vi "UHR-Fleezers Control (host) - Avogadro v2.vi"() -> ()   [LabVIEW 2014] (continued)
0.06928382213812578, 0.06928028199102658, 0.06922544022949823, 0.06920560319833882, 0.06922019104586834, 0.06924063844721727, 0.06926700643940453, 0.06926718955046138, 0.06929898983733536, 0.06925055696279696, 0.06931403546250704, 0.0692955107272551, 0.06922473830378026, 0.06928565324869435, 0.06928879665517038, 0.06925675222022058, 0.06923380230109463, 0.06924164555802997, 0.06928174687948142, 0.06932566301461739, 0.06929343546861073, 0.06929117709890951, 0.06922135074922843, 0.06925714896084378, 0.06925159459211913, 0.06932630390331637, 0.0692147892696911, 0.0692787255470433, 0.06924900051881369, 0.06927286599322391, 0.06931833857234315, 0.06929380169072444, 0.06926581621753496, 0.06930823694570659, 0.06927799310281588, 0.06928147221289614, 0.06926407666249483, 0.06927030243842792, 0.06922562334055508, 0.06926313058870108, 0.06927741325113584, 0.06928653828546916, 0.0692268440809341, 0.06926950895718155, 0.06926767784661299, 0.06920160527359746, 0.06925424970244355, 0.06928284554582255, 0.06921207312234773, 0.06924927518539896, 0.06922894985808796, 0.0692571184423343, 0.06920566423535776, 0.06925980407116819, 0.06928257087923728, 0.06927216406750597, 0.06922339548936332, 0.06926215399639785, 0.06920325327310915, 0.06924637592699874, 0.06921677297280703, 0.06922513504440345, 0.06916922513504342, 0.06923242896816821, 0.06922205267494637, 0.06921817682424293, 0.06918747520371007, 0.06919815668202667, 0.06919797357096982, 0.06923786126285494, 0.06921915341654616, 0.06922568437757402, 0.06918127994628644, 0.06922547074800768, 0.06924582659382818, 0.06921549119540904, 0.0692108218634592, 0.06915109714041469, 0.06908627582628768, 0.06918482009338565, 0.0691833857234403, 0.06921112704855398, 0.06916605121005792, 0.06920618305001885, 0.069132267220068, 0.06920310068056178, 0.06923773918881705, 0.06922501297036555, 0.0691231116672252, 0.06918146305734331, 0.06919553209021173, 0.06922956022827748, 0.06919336527603893, 0.06926355784783372, 0.06923966185491404, 0.06929560228278353, 0.06927195043793963, 0.06928467665639111, 0.06924256111331427, 0.06929725028229522, 0.06923395489364202, 0.06924204229865316, 0.06922525711844135, 0.06924771874141569, 0.06915643787957299, 0.06924536881618604, 0.06916010010071011, 0.06918335520493081, 0.06919299905392522, 0.06916858424634442, 0.06912195196386511, 0.06918533890804675, 0.06917004913479928, 0.0691453596606332, 0.06913382366405128, 0.06916522721030208, 0.06916882839442023, 0.06921610156559856, 0.06917017120883717, 0.0692243110446476, 0.06924466689046808, 0.06922168645283266, 0.06920572527237671, 0.06918127994628644, 0.06914984588152617, 0.06918936735129759, 0.06918237861262758, 0.0692385631885729, 0.06924268318735215, 0.06924527726065761, 0.06918936735129759, 0.06917838068788623, 0.0691982482375551, 0.06920844141972009, 0.06918158513138122, 0.06920218512527751, 0.06922443311868551, 0.06925321207312136, 0.06926328318124844, 0.06932975249488717, 0.0693037812433231, 0.06932642597735428, 0.06933487960447914, 0.0693373516037467, 0.06928443250831531, 0.0693576769310577, 0.06930802331614026, 0.06936115604113798, 0.06934812463759171, 0.06937299722281466, 0.06932422864467201, 0.0693681142612985, 0.06933906064027735, 0.0693524582659373, 0.06936597796563516, 0.06941334269234192, 0.0694059877315582, 0.0694610431226529, 0.06942216254158048, 0.06946394238105313, 0.06943000579851583, 0.06939817499313235, 0.06938685262611675, 0.06938254951628064, 0.06940998565629956, 0.06944059572130398, 0.06940183721426947, 0.06945286416211334, 0.06943455305642773, 0.06941611987670424, 0.06938065736869313, 0.06938911099581799, 0.06940125736258942, 0.06936140018921379, 0.06936152226325168, 0.06936069826349583, 0.06934803308206329, 0.06941767632068752, 0.06940769676808886, 0.06943382061220031, 0.06938242744224274, 0.06941331217383244, 0.06935120700704879, 0.06939872432630292, 0.06936268196661176, 0.06943717764824267, 0.06937897885067196, 0.06938016907254152, 0.06935740226447241, 0.0693983581041892, 0.06941715750602642, 0.0694203619495214, 0.06937653736991388, 0.06944013794366186, 0.0693949400311279, 0.06943995483260498, 0.06938178655354375, 0.0694314096499517, 0.06938126773888265, 0.06940684224982353, 0.06935407574693954, 0.06939741203039546, 0.06940458388012231, 0.06944648579363286, 0.06942982268745895, 0.06944026001769976, 0.06939869380779344, 0.0694128543961903, 0.06941743217261172, 0.0694466689046897, 0.06944306772057154, 0.06944724875636975, 0.0693813287759016, 0.0694225287636942, 0.06942335276345005, 0.06942286446729842, 0.06936649678029627, 0.06939878536332188, 0.06938465529343447, 0.06938209173863849, 0.06943617053742997, 0.06940986358226166, 0.0693832514419986, 0.06940720847193725, 0.06944444105349797, 0.06941395306253144, 0.06938648640400304, 0.0693665883358247, 0.06930732139042231, 0.0692876369518103, 0.06930552079836323, 0.06935331278420263, 0.0692883999145472, 0.06935364848780687, 0.06931913205358953, 0.06933057649464301, 0.06932050538651595, 0.0692761925107568, 0.0693024994659251, 0.06931672109134092, 0.06930591753898642, 0.06935569322794176, 0.06926532792138335, 0.06928382213812578, 0.06927756584368322, 0.06927701651051264, 0.06923596911526743, 0.06926230658894522, 0.06935776848658613, 0.06929181798760851, 0.06931965086825062, 0.06932584612567425, 0.06934714804528849, 0.06931525620288607, 0.06937565233313907, 0.06932847071748918, 0.06936109500411901, 0.06931763664662519, 0.0692788476210812, 0.06924845118564311, 0.06926844080934988, 0.06921359904782153, 0.06921311075166992, 0.06931092257454047, 0.0693307290871904, 0.06935657826471657, 0.06931730094302097, 0.0693545030060722, 0.06926172673726516, 0.06934031189916587, 0.06935810419019038, 0.06938956877346013, 0.06931397442548808, 0.06935932493056941, 0.06935944700460732, 0.06934925382244232, 0.06938404492324496, 0.06937766655476449, 0.06930881679738664, 0.06933249916074001, 0.06928376110110684, 0.06932816553239442, 0.06931122775963525, 0.06934678182317477, 0.06935254982146573, 0.06938245796075221, 0.06937485885189269, 0.06939579454939322, 0.06931440168462075, 0.06936371959593396, 0.06932306894131193, 0.06934836878566752, 0.0693476363414401, 0.06934827723013909, 0.06930079042939444, 0.06931440168462075, 0.06926267281105893, 0.06928592791527964, 0.0692700888088616, 0.06928601947080806, 0.06929694509720048, 0.06930405590990837, 0.06929740287484261, 0.06930442213202209, 0.06922742393261415, 0.06928464613788164, 0.0692596514786208, 0.06930793176061184, 0.069199652088991, 0.06925479903561411, 0.06921405682546367, 0.06921103549302554, 0.0692374340037223, 0.0692571184423343, 0.06916357921079036, 0.06923007904293857, 0.06926007873775347, 0.06929618213446358, 0.06919635608996759, 0.06923010956144804, 0.06919727164525186, 0.06923825800347815, 0.06919989623706681, 0.06925031281472116, 0.06920294808801442, 0.06928122806482033, 0.06922745445112363, 0.06929078035828631, 0.06922525711844137, 0.06926862392040675, 0.06922998748741013, 0.06929773857844684, 0.06921878719443245, 0.0692302926725049, 0.06921588793603223, 0.06924692526016932, 0.06919693594164764, 0.0692117374187435, 0.06916132084108916, 0.0692548295541236, 0.06917160557878256, 0.06922321237830648, 0.06927637562181364, 0.06926190984832203, 0.06919534897915489, 0.0692418591875963, 0.06920361949522287, 0.06919110690633773, 0.06915567491683608, 0.06916843165379705, 0.06909604174932, 0.0691276894436466, 0.06915414899136228, 0.06914127018036341, 0.06910113834040249, 0.06911123996703905, 0.0691143528550056, 0.06914590899380377, 0.06910333567308476, 0.06913177892391639, 0.0690913418988607, 0.06912509537034113, 0.06914682454908805, 0.06910397656178374, 0.06911520737327093, 0.06913068025757525, 0.06910980559709366, 0.06910458693197327, 0.06907867671742815, 0.06909610278633894, 0.06905011139255862, 0.06911847285378485, 0.0691039155247648, 0.0691266823328339, 0.06910153508102568, 0.06914807580797655, 0.06916101565599438, 0.06917352824487955, 0.06917227698599103, 0.0691720633564247, 0.06911679433576366, 0.06917352824487955, 0.06914658040101224, 0.06918637653736893, 0.06920084231086056, 0.06919824823755509, 0.06915613269447822, 0.06918848231452278, 0.06918335520493081, 0.06919895016327304, 0.06913116855372686, 0.0691971190527045, 0.06918787194433326, 0.06919757683034664, 0.06918262276070339, 0.06924823755607679, 0.06920020142216156, 0.06926316110721055, 0.06924225592821949, 0.06923294778282932, 0.06919544053468331, 0.06923789178136441, 0.06921427045503001, 0.06923743400372227, 0.06922196111941795, 0.06923917355876243, 0.06915729239783831, 0.06921027253028865, 0.06919714957121396, 0.0692110965300445, 0.06918735312967217, 0.06918729209265322, 0.06915085299233888, 0.06920081179235107, 0.06917542039246705, 0.06917288735618055, 0.0691332743308807, 0.06919083223975243, 0.06917096469008356, 0.06918506424146147, 0.06919516586809803, 0.06922379222998651, 0.06913037507248047, 0.06924118778038783, 0.06920123905148376, 0.06923831904049708, 0.06914429151280153, 0.06924344615008905, 0.06921396526993524, 0.06924512466811023, 0.06916586809900106, 0.06923044526505227, 0.0691588488418216, 0.06921011993774126, 0.06913885921811481, 0.06914893032624188, 0.0691214636677135, 0.06917664113284609, 0.06917542039246706, 0.06919003875850606, 0.0692187261574135, 0.06922055726798206, 0.06918701742606793, 0.06921475875118162, 0.06920477919858296, 0.06921805475020502, 0.06920517593920615, 0.06922910245063534, 0.06923438215277468, 0.06924124881740677, 0.06926117740409461, 0.06928516495254274, 0.06921857356486612, 0.06925373088778247, 0.06925061799981592, 0.06924826807458626, 0.0692750328073967, 0.06931464583269656, 0.06937162388988824, 0.06935654774620709, 0.06929197058015589, 0.06936548966948355, 0.0693017365031882, 0.06939542832727952, 0.06935874507888937, 0.06938279366435644, 0.06938038270210783, 0.06944230475783464, 0.06940006714071986, 0.06944495986815905, 0.06940940580461952, 0.0694348582415225, 0.06944514297921592, 0.0694868617816696, 0.06947965941343326, 0.06947242652668745, 0.06950325022125821, 0.06952189703054804, 0.0694953764458134, 0.06957673879207642, 0.06949229407635632, 0.06953450117496163, 0.06946507156590373, 0.06954097109897055, 0.06946720786156706, 0.0694868617816696, 0.06952623065889363, 0.06954994354075647, 0.06957148960844654, 0.06959816278572856, 0.0695725577562782, 0.06958680990020348, 0.06958510086367282, 0.06966365550706405, 0.06963698232978202, 0.06965819269386785, 0.06967076631977195, 0.0697335123752546, 0.06973534348582316, 0.06974614703817766, 0.06976375621814532, 0.06982854701376286, 0.06980843531601817, 0.06983645130771712, 0.06984640034180632, 0.0698301339762556, 0.06985320596941946, 0.06992004150517189, 0.06990957365642161, 0.06995046845911945, 0.06997314371166012, 0.06997930845057428, 0.0699218115787215, 0.06998873867000237, 0.06995327616199125, 0.06998364207891987, 0.06994909512619303, 0.06998275704214507, 0.06993319498275605, 0.06996145512253081, 0.06991296121097346, 0.06991021454512061, 0.06985512863551643, 0.06990252388073266, 0.06985839411603037, 0.06987047944578287, 0.06978942228461463, 0.06983977782525001, 0.06983184301278626, 0.06985430463576059, 0.06982995086519875, 0.0698108157597573, 0.06970448927274292, 0.06973931089205504, 0.06972115237891682, 0.06972475356303498, 0.06966628009887897, 0.06968923001800492, 0.06967735831781877, 0.06963875240333163, 0.0696143681142603, 0.06966029847102168, 0.0695813165684978, 0.06959044160283114, 0.06961366618854235, 0.06961302529984337, 0.06952928250984124, 0.06950944547868183, 0.06949415570543435, 0.06950706503494271, 0.06950004577776323, 0.06943632312997734, 0.0693612475966664, 0.06943348490859608, 0.06937556077761065, 0.0694244209112817, 0.06940198980681685, 0.06936371959593396, 0.0694281136509283, 0.06942793053987145, 0.06935752433851032, 0.0694109622486028, 0.06932496108889943, 0.06942591631824603, 0.06935749382000085, 0.06932734153263857, 0.06933256019775896, 0.06936927396465858, 0.06926697592089504, 0.06920108645893637, 0.06925611133152158, 0.069275307473982, 0.06927207251197755, 0.0692443006683544, 0.06925595873897421, 0.06922525711844135, 0.06900939970091766, 0.06908078249458201, 0.06901355021820639, 0.06906955168309484, 0.06910080263679826, 0.06912570574053066, 0.06909518723105468, 0.06909280678731554, 0.0690646382030692, 0.06911597033600783, 0.06913183996093533, 0.06914200262459085, 0.06908282723471688, 0.06905606250190645, 0.06909497360148835, 0.06913501388592083, 0.06918384350108242, 0.0692108218634592, 0.06919464705343693, 0.06925086214789171, 0.06925498214667097, 0.06924631488997979, 0.06922464674825184, 0.06922428052613812, 0.0691827448347413, 0.06927976317636549, 0.06925122837000543, 0.06928266243476572, 0.06925428022095302, 0.06927176732688277, 0.06923767815179808, 0.06924048585466987, 0.06918768883327642, 0.06921976378673568, 0.06917627491073237, 0.06922287667470223, 0.06926493118076016, 0.06929166539506112, 0.0692335886715283, 0.06928254036072781, 0.0693138218329407, 0.06933661915951927, 0.06939020966215913, 0.06940009765922935, 0.06936078981902426, 0.06939298684652143, 0.06944074831385137, 0.06944294564653364, 0.06942085024567303, 0.06943821527756486, 0.06940995513779008, 0.06946574297311221, 0.06951628162480446, 0.06949946592608319, 0.06942378002258272, 0.06949400311288698, 0.06946589556565959, 0.06944950712607098, 0.06951783806878772, 0.06949861140781786, 0.0694629657887499, 0.06952259895626599, 0.0695176244392214, 0.06947825556199737, 0.06942573320718919, 0.06947831659901632, 0.06941587572862842, 0.06947450178533181, 0.06938346507156493, 0.06943455305642773, 0.06940266121402533, 0.06944734031189818, 0.06939082003234864, 0.06941593676564738, 0.06940067751090938, 0.0694282357249662, 0.06941657765434639, 0.06942674031800189, 0.06941163365581127, 0.06939527573473213, 0.06937739188817921, 0.06944236579485359, 0.06937946714682357, 0.06939136936551919, 0.06931134983367315, 0.06937668996246125, 0.0693743400372316, 0.06936866359446905, 0.06935389263588268, 0.06936960966826282, 0.06930698568681808, 0.06940647602770983, 0.0693743400372316, 0.06936530655842671, 0.0693283181249418, 0.06937260048219147, 0.06928708761863972, 0.06929853205969323, 0.06928260139774675, 0.06927167577135435, 0.06921579638050379, 0.06923749504074124, 0.06932084109012018, 0.0692972808008047, 0.06927115695669325, 0.06927240821558178, 0.06923496200445473, 0.06923291726431982, 0.0692414624469731, 0.06924652851954613, 0.06924222540971, 0.06927967162083705, 0.06922196111941795, 0.0692802514725171, 0.06921662038025965, 0.06925281533249818, 0.06915695669423408, 0.06924216437269105, 0.06919656971953392, 0.06922272408215485, 0.06905246131778828, 0.06903219702749622, 0.06897784356211946, 0.06902172917874595, 0.06904290902432228, 0.06901373332926324, 0.0689079866939289, 0.06895702993865684, 0.06897759941404365, 0.06904547257911826, 0.06898510696737475, 0.06900979644154083, 0.06893527024140045, 0.06896411023285527, 0.06895205542161224, 0.06902035584581953, 0.06896182134464457, 0.0689088717307037, 0.0689659718619333, 0.06894393749809163, 0.06894552446058438, 0.06899407940916069, 0.06902359080782398, 0.06900610370189425, 0.06896398815881737, 0.06897000030518413, 0.06895303201391548, 0.06892394787438486, 0.06891708120975276, 0.06895614490188204, 0.06893386638996456, 0.06896029541917077, 0.06893047883541271, 0.06892196417126892, 0.0688969389934986, 0.06887713248084867, 0.06886898403881858, 0.06889373455000361, 0.06893179113132018, 0.0689844050416568, 0.06896029541917077, 0.06903549302651962, 0.06898696859645279, 0.06904702902310154, 0.06897976622821646, 0.06901742606890983, 0.06895489364299351, 0.06902398754844717, 0.06895928830835805, 0.06899652088991877, 0.06892529068880181, 0.06907742545853965, 0.0689923093356111, 0.06904068117313054, 0.06901293984801687, 0.0690629902035575, 0.06898751792962336, 0.06905212561418404, 0.06901574755088866, 0.06903057954649398, 0.06902786339915062, 0.06900390636921197, 0.06897775200659104, 0.06903225806451517, 0.06900073244422647, 0.06899374370555646, 0.06898916592913507, 0.06902673421430001, 0.06899829096346839, 0.06899816888943049, 0.06897946104312169, 0.0689425946836747, 0.06894210638752307, 0.06898773155918968, 0.06898156682027555, 0.06902923673207703, 0.0690891750846879, 0.06910986663411262, 0.06898773155918968, 0.06899493392742602, 0.06893603320413735, 0.06897277748954646, 0.0689700308236936, 0.06903515732291539, 0.06900006103701799, 0.06902288888210603, 0.06905810724204134, 0.06907666249580274, 0.0690476088747816, 0.06911822870570904, 0.06903579821161439, 0.06912289803765886, 0.06906640827661881, 0.06910397656178374, 0.0690969267860948, 0.06909479049043148, 0.06906573686941032, 0.06907480086672471, 0.06907513657032893, 0.06911139255958643, 0.06906640827661881, 0.06908938871425423, 0.06898767052217074, 0.06905703909420968, 0.06905963316751514, 0.06907953123569348, 0.06908258308664109, 0.06913657032990411, 0.0691284524063835, 0.06918887905514597, 0.06916141239661758, 0.06918411816766772, 0.0690843531601907, 0.06914716025269228, 0.06917557298501444, 0.06914508499404792, 0.06910473952452065, 0.0691471297341828, 0.06909408856471352, 0.06915491195409917, 0.06904681539353522, 0.06899890133365791, 0.06896469008453532, 0.06900885036774708, 0.06898336741233461, 0.0690029602954182, 0.06898751792962336, 0.06901153599658096, 0.06898599200414955, 0.06896377452925104, 0.06896636860255649, 0.0689640491958363, 0.06888872951444955, 0.06892983794671373, 0.06889773247474497, 0.06892974639118529, 0.06884310434278294, 0.0688693502609323, 0.06882906582842398, 0.06887527085177064, 0.06881289101840171, 0.06882760093996913, 0.06880477309488109, 0.06884682760093902, 0.06882729575487438, 0.06880715353862021, 0.06879787591173951, 0.06876665547654556, 0.06877254554887444, 0.0688024842066704, 0.0687996765037986, 0.06876290169988003, 0.06870812097537062, 0.06874761192663255, 0.06874776451917992, 0.06873366496780202, 0.06870973845637283, 0.06873259681997035, 0.06870989104892021, 0.06874285103915428, 0.06875408185064145, 0.06876287118137055, 0.06868306527909082, 0.0687413251136805, 0.06873516037476633, 0.06876705221716876, 0.06874877162999264, 0.06876073488570723, 0.06875914792321448, 0.0687666249580361, 0.0687452620014029, 0.06872701193273625, 0.06869734794152559, 0.06874620807519666, 0.06871886349070616, 0.06876186407055784, 0.06878420361949426, 0.06878331858271947, 0.0687811212500372, 0.06880874050111296, 0.06880281991027462, 0.06881554612872612, 0.06877559739982204, 0.06879134495071165, 0.06878319650868157, 0.06880166020691454, 0.06881356242561018, 0.06884148686178071, 0.06881026642658677, 0.06884322641682085, 0.06880458998382423, 0.06882033753471385, 0.06878203680532147, 0.06879219946897698, 0.06879708243049314, 0.0688984649189724, 0.06890578936124664, 0.06884621723074949, 0.06881997131260013, 0.06891769157994228, 0.06881914731284428, 0.06874419385357124, 0.06876387829218325, 0.06874108096560469, 0.06872273934140961, 0.06871807000945979, 0.06872405163731707, 0.06872469252601608, 0.0687376323740339, 0.06876287118137055, 0.06875310525833822, 0.06868214972380654, 0.06878228095339728, 0.0687132175664531, 0.06875292214728138, 0.06875737784966486, 0.06874391918698596, 0.06877846613971278, 0.06878829309976406, 0.06880794701986659, 0.06870842616046537, 0.06872151860103057, 0.06874398022400491, 0.06877193517868492, 0.06870815149388008, 0.06875981933042294, 0.06872319711905174, 0.06876705221716876, 0.06879403057954554, 0.06886315500350867, 0.06883440656758227, 0.06884914700765919, 0.06886785485396797, 0.06886223944822438, 0.06883373516037382, 0.0688524430066826, 0.06879424420911187, 0.06881069368571943, 0.0688163396099725, 0.06889284951322881] caption="Most Recent Time Trace"
  out "Values":dbl[](array[numeric])=[0.020926881619989478, 0.0011467646305518288, 2.9154516281624803, -0.030429562905799058, -0.00042677435028031413, 2.950325037385175, -0.06640585647249925, 1.9997715994750818, -0.2051950626816138, 1.999770470290231, -0.03222110241124139, -0.03281923296074719, 2.4438679006317336]
  out "All Signals":waveform(dbl)[](graph)=[{"t0"=timestamp(907.4000000000693 s since 1904-01-01), "dt"=0.15, "Y"=[0.0], "attributes"=variant("NI_ChannelName"=variant(string "APD 1"))}, {"t0"=timestamp(907.4000000000693 s since 1904-01-01), "dt"=0.15, "Y"=[0.0], "attributes"=variant("NI_ChannelName"=variant(string "APD 2"))}, {"t0"=timestamp(907.4000000000693 s since 1904-01-01), "dt"=0.15, "Y"=[0.0], "attributes"=variant("NI_ChannelName"=variant(string "APD 3"))}, {"t0"=timestamp(907.4000000000693 s since 1904-01-01), "dt"=0.1, "Y"=[0.0209008038928622, 0.020952959347116742], "attributes"=variant("NI_ChannelName"=variant(string "T1 Y"))}, {"t0"=timestamp(907.4000000000693 s since 1904-01-01), "dt"=0.1, "Y"=[0.0011049463527954713, 0.0011885829083081864], "attributes"=variant("NI_ChannelName"=variant(string "T1 X"))}, {"t0"=timestamp(907.4000000000693 s since 1904-01-01), "dt"=0.1, "Y"=[2.9152944120609123, 2.9156088442640438], "attributes"=variant("NI_ChannelName"=variant(string "T1 Sum"))}, {"t0"=timestamp(907.4000000000693 s since 1904-01-01), "dt"=0.1, "Y"=[-0.0304555117085528, -0.030403614103045283], "attributes"=variant("NI_ChannelName"=variant(string "T2 Y"))}, {"t0"=timestamp(907.4000000000693 s since 1904-01-01), "dt"=0.1, "Y"=[-0.0004450976345029815, -0.0004084510660576463], "attributes"=variant("NI_ChannelName"=variant(string "T2 X"))}, {"t0"=timestamp(907.4000000000693 s since 1904-01-01), "dt"=0.1, "Y"=[2.9503227637562124, 2.950327311014123], "attributes"=variant("NI_ChannelName"=variant(string "T2 Sum"))}, {"t0"=timestamp(907.4000000000693 s since 1904-01-01), "dt"=0.1, "Y"=[-0.06637311145084834, -0.06643860149415003], "attributes"=variant("NI_ChannelName"=variant(string "T1 FB X"))}, {"t0"=timestamp(907.4000000000693 s since 1904-01-01), "dt"=0.1, "Y"=[1.9997719046601732, 1.9997712942899846], "attributes"=variant("NI_ChannelName"=variant(string "T1 FB Sum"))}, {"t0"=timestamp(907.4000000000693 s since 1904-01-01), "dt"=0.1, "Y"=[-0.20517833433578245, -0.20521179102744508], "attributes"=variant("NI_ChannelName"=variant(string "T2 FB X"))}, {"t0"=timestamp(907.4000000000693 s since 1904-01-01), "dt"=0.1, "Y"=[1.9997702261421568, 1.9997707144383057], "attributes"=variant("NI_ChannelName"=variant(string "T2 FB Sum"))}, {"t0"=timestamp(907.4000000000693 s since 1904-01-01), "dt"=0.1, "Y"=[-0.03224579759693241, -0.03219640722555035], "attributes"=variant("NI_ChannelName"=variant(string "T3 Y/ PSD Y"))}, {"t0"=timestamp(907.4000000000693 s since 1904-01-01), "dt"=0.1, "Y"=[-0.0328433863084647, -0.0327950796130297], "attributes"=variant("NI_ChannelName"=variant(string "T3 X / PSD X"))}, {"t0"=timestamp(907.4000000000693 s since 1904-01-01), "dt"=0.1, "Y"=[2.4440564592425247, 2.443679342020927], "attributes"=variant("NI_ChannelName"=variant(string "T3 Sum / PSD sum"))}]
  in  "Signals to Plot":i32(listbox)=7
  out "Trap Disp. Freq. (Hz)":dbl=10.0 caption="Freq. (Hz)" format="%#_6p"
  out "Display Period (s)":dbl=0.1 caption="Period (s)" format="%#_6p"
  in  "Trap Disp. Downsample":dbl=10000.0 caption="Downsample" max=20000.0
  in  "APD Disp. Scale":dbl=0.1 caption="Scale (Divide,\nfor above plot only)"
  in  "APD Disp. Downsample":dbl=150.0 caption="Integrate" max=200.0
  out "APD Display Freq. (Hz)":dbl=6.666666666666667 caption="Freq. (Hz)"
  out "APD Display Period (s)":dbl=0.15 caption="Period (s)"
  out "FFT 1":cluster{"f0":dbl, "df":dbl, "magnitude":dbl[]}[](graph)=[{"f0"=0.0, "df"=3.3333333333333335, "magnitude"=array[10000 elements]}, {"f0"=0.0, "df"=3.3333333333333335, "magnitude"=array[10000 elements]}]
  out "FFT 2":cluster{"f0":dbl, "df":dbl, "magnitude":dbl[]}[](graph)
  in  "FFT 1 Choice 1":u16(ring) items=["T1 Y", "T1 X", "T1 Sum", "T2 Y", "T2 X", "T2 Sum", "T1 FB X", "T1 FB Sum", "T2 FB X", "T2 FB Sum", "PSD Y", "PSD X", "PSD Y Sum", "none"]
  in  "FFT 2 Choice 1":u16(ring)=13 items=["T1 Y", "T1 X", "T1 Sum", "T2 Y", "T2 X", "T2 Sum", "T1 FB X", "T1 FB Sum", "T2 FB X", "T2 FB Sum", "PSD Y", "PSD X", "PSD Y Sum", "none"]
  in  "FFT 1 Choice 2":u16(ring)=1 items=["T1 Y", "T1 X", "T1 Sum", "T2 Y", "T2 X", "T2 Sum", "T1 FB X", "T1 FB Sum", "T2 FB X", "T2 FB Sum", "PSD Y", "PSD X", "PSD Y Sum", "none"]
  in  "FFT 2 Choice 2":u16(ring)=13 items=["T1 Y", "T1 X", "T1 Sum", "T2 Y", "T2 X", "T2 Sum", "T1 FB X", "T1 FB Sum", "T2 FB X", "T2 FB Sum", "PSD Y", "PSD X", "PSD Y Sum", "none"]
  in  "Compute FFT":bool
  in  "Reset FFT":bool
  in  "# Spectra to Ave.":dbl=25.0
  out "Ave. Time (s)":dbl=7.5
  out "1 Channel":waveform(dbl)(graph)={"t0"=timestamp(0 s since 1904-01-01), "dt"=1e-05, "Y"=array[20000 elements], "attributes"=variant("NI_ChannelName"=variant(string "T1 X"))}
  out "Slow mean":dbl=0.0011467646305518288 format="%0.2f"
  in  "Slow mean N ave.":dbl=1.0 min=1.0 step=1.0
  out "Mean Intensity":dbl=0.0011467646305518293
  out "Sigma":dbl=0.00034701935250238753
  out "Sigma/Mean":dbl=0.30260730341447656
  in  "Subtract mean":bool
  in  "High Res. Display":u16(ring)=1 items=["T1 Y", "T1 X", "T1 Sum", "T2 Y", "T2 X", "T2 Sum", "T1 FB X", "T1 FB Sum", "T2 FB X", "T2 FB Sum", "PSD Y", "PSD X", "PSD Y Sum"]
  out "Output Means":T9={"Ext1 (nm)"=2762.837091578119, "F1 pN)"=12.13669896208951, "Ext 2 (nm)"=310.7072373075949, "F2 (pN)"=16.26099481300423, "Ext 3 (nm)"=926.7829395108193, "Numeric 6"=18.116447924023788}
  out "tether forces":waveform(dbl)[](graph)=[{"t0"=timestamp(907.4000000000693 s since 1904-01-01), "dt"=0.1, "Y"=[12.13150652795135, 12.141891396227669], "attributes"=variant("NI_ChannelName"=variant(string "Tether 1"))}, {"t0"=timestamp(907.4000000000693 s since 1904-01-01), "dt"=0.1, "Y"=[16.262549777040206, 16.259439848968256], "attributes"=variant("NI_ChannelName"=variant(string "Tether 2"))}, {"t0"=timestamp(907.4000000000693 s since 1904-01-01), "dt"=0.1, "Y"=[18.11722029082963, 18.115675557217948], "attributes"=variant("NI_ChannelName"=variant(string "Tether 3"))}]
  out "2D tethers":waveform(dbl)[](graph)=[{"t0"=timestamp(907.4000000000693 s since 1904-01-01), "dt"=0.1, "Y"=[2768.869200345611, 2756.804982810627], "attributes"=variant("NI_ChannelName"=variant(string "Tether 1"))}, {"t0"=timestamp(907.4000000000693 s since 1904-01-01), "dt"=0.1, "Y"=[305.6847282884945, 315.72974632669525], "attributes"=variant("NI_ChannelName"=variant(string "Tether 2"))}, {"t0"=timestamp(907.4000000000693 s since 1904-01-01), "dt"=0.1, "Y"=[932.9253246765345, 920.6405543451042], "attributes"=variant("NI_ChannelName"=variant(string "Tether 3"))}]
  out "2D forces":waveform(dbl)[](graph)=[{"t0"=timestamp(907.4000000000693 s since 1904-01-01), "dt"=0.1, "Y"=[10.809672659724802, 10.828889591681625], "attributes"=variant("NI_ChannelName"=variant(string "Trap 1 X"))}, {"t0"=timestamp(907.4000000000693 s since 1904-01-01), "dt"=0.1, "Y"=[-5.506761991163622, -5.491873713857308], "attributes"=variant("NI_ChannelName"=variant(string "Trap 1 Y"))}, {"t0"=timestamp(907.4000000000693 s since 1904-01-01), "dt"=0.1, "Y"=[12.364602742140338, 12.37322540337601], "attributes"=variant("NI_ChannelName"=variant(string "Trap 2 X"))}, {"t0"=timestamp(907.4000000000693 s since 1904-01-01), "dt"=0.1, "Y"=[-10.563480689610127, -10.548586508128349], "attributes"=variant("NI_ChannelName"=variant(string "Trap 2 Y"))}, {"t0"=timestamp(907.4000000000693 s since 1904-01-01), "dt"=0.1, "Y"=[11.437990795248211, 11.44891346548756], "attributes"=variant("NI_ChannelName"=variant(string "Trap 3 X"))}, {"t0"=timestamp(907.4000000000693 s since 1904-01-01), "dt"=0.1, "Y"=[-14.050125893893833, -14.039233645543526], "attributes"=variant("NI_ChannelName"=variant(string "Trap 3 Y"))}]
  in  "2D force calibration":u16(ring)=2 items=["None", "Position", "Force"]
  out "Positions \nand displacements":cluster{"X":dbl[], "Y":dbl[]}[](graph)=[{"X"=[2029.9999999999682, 2029.9999999999682], "Y"=[0.0, 0.0]}, {"X"=[6090.0, 6090.0], "Y"=[0.0, 0.0]}, {"X"=[3856.3118985290066, 3856.3118985290066], "Y"=[-2.7867843867294573, -2.7867843867294573]}, {"X"=[2029.9999999999682, 2544.8742933601216, 2545.78961286824], "Y"=[0.0, -258.0585274124136, -257.36083121208026]}, {"X"=[6090.0, 6672.642343132017, 6673.048658454163], "Y"=[0.0, -495.20546004269727, -494.5072356402143]}, {"X"=[3856.3118985290066, 4572.072258702311, 4572.7557716133215], "Y"=[-2.7867843867294573, -946.7988381703877, -946.0670003339764]}, {"X"=[12068.90144948506, 12068.90144948506], "Y"=[-5102.478497055473, -5102.478497055473]}, {"X"=[5138.691126639824, 5138.691126639824], "Y"=[-1579.9076458090763, -1579.9076458090763]}, {"X"=[-1258.8588574892046, -1258.8588574892046], "Y"=[6271.8884837027335, 6271.8884837027335]}, {"X"=[5316.244572878561, 5316.244572878561], "Y"=[-136.83255305393848, -136.83255305393848]}]
  in  "Measure \ncorrelation?":bool
  out "AOM position for scan (MHz)":dbl=80.0
  in  "Stop scan":bool
  out "Position\nscanning...":bool
  in  "Start position \nscan":bool
  out "Correlations in Y":dbl[][](graph)
  out "Correlations in X":dbl[][](graph)
  out "3-1 x correlation":dbl=-1.1268659629352283e-07
  out "3-1 y correlation":dbl=-7.943511528650863e-08
  in  "Correlation integration time (s)":dbl=0.2
  in  "T3 positioning test range (V)":T10={"Xmin"=3.6, "Xmax"=5.21, "Ymin"=0.5, "Ymax"=2.11, "increment"=0.1}
  in  "Tab Control":T11(tab)=enum."Misc. Configuration"
  in  "Shift offset":bool
  in  "Scaling factor":dbl=0.25
  in  "Scale intensities":bool
  in  "Trap 3 Bead Size (nm)":dbl=1000.0
  in  "T3 calibration":T12={"alpha_x (nm/V)"=707.4722301487932, "offset_x (mV)"=-83.42914287044084, "kappa_x (pN/nm)"=0.319603918620997, "alpha_y (nm/V)"=740.8709591900941, "kappa_y (pN/nm)"=0.29766835788971263, "offset_y (mV)"=31.463816207854467} {"offset_y (mV)" format="%#_2g"; "kappa_y (pN/nm)" min=0.0 step=0.001 format="%#_2g"; "alpha_y (nm/V)" step=10.0 format="%#_3g"; "kappa_x (pN/nm)" min=0.0 step=0.001 format="%#_2g"; "offset_x (mV)" format="%#_2g"; "alpha_x (nm/V)" step=10.0 format="%#_3g"}
  in  "T2 calibration":T12={"alpha_x (nm/V)"=554.3702171630429, "offset_x (mV)"=-52.99502952962309, "kappa_x (pN/nm)"=0.42443199976417534, "alpha_y (nm/V)"=672.6942367136504, "kappa_y (pN/nm)"=0.42663021884691377, "offset_y (mV)"=6.352107044207092} {"offset_y (mV)" format="%#_2g"; "kappa_y (pN/nm)" min=0.0 step=0.001 format="%#_2g"; "alpha_y (nm/V)" step=10.0 format="%#_3g"; "kappa_x (pN/nm)" min=0.0 step=0.001 format="%#_2g"; "offset_x (mV)" format="%#_2g"; "alpha_x (nm/V)" step=10.0 format="%#_3g"}
  in  "Visa resource for valves":refnum<visa-resource-name>="COM3"
  in  "Cursor control":cluster{"X":bool, "Y":bool}
  in  "Trap 3 (ON/OFF)":bool=TRUE
  in  "Maximum Delta\n(MHz)":dbl=30.0
  in  "T3 Y (V)":dbl=1.24 min=0.0 max=10.0 step=1.0 format="%#_6f"
  in  "T3 X (V)":dbl=4.32 min=0.0 max=10.0 step=1.0 format="%#_6f"
  in  "Shunt 1":bool caption="Inject Pump 3"
  in  "manual raster set":u16(ring) items=["offset", "user-defined", "basepaire step", "user-defined 2", "user-defined 3", "user-defined 4"]
  in  "move Con X?":bool
  in  "Symmetric?":bool
  out "Laser Intensity Low (bugs to fix)":bool
  out "Good freq?":bool=TRUE
  in  "T1 calibration":T12={"alpha_x (nm/V)"=547.2006244799962, "offset_x (mV)"=-45.94126214243769, "kappa_x (pN/nm)"=0.4198956055537018, "alpha_y (nm/V)"=668.8621643752366, "kappa_y (pN/nm)"=0.42678395838189426, "offset_y (mV)"=40.191663890411775} {"offset_y (mV)" format="%#_2g"; "kappa_y (pN/nm)" min=0.0 step=0.001 format="%#_2g"; "alpha_y (nm/V)" step=10.0 format="%#_3g"; "kappa_x (pN/nm)" min=0.0 step=0.001 format="%#_2g"; "offset_x (mV)" format="%#_2g"; "alpha_x (nm/V)" step=10.0 format="%#_3g"}
  in  "Blue FB Setpoint (mV)":dbl=90.0
  in  "Blue Laser ON":bool
  in  "11":bool
  out "Stage Moving":bool
  in  "Read Cal":bool
  in  "Speed (nm/s)":dbl=100.0
  in  "Furthest Withdraw (MHz)":dbl=15.0
  in  "Round T1 X":bool caption="Round"
  in  "Cal sets to save":u32=25 min=1 step=1
  in  "Trap 2 (ON/OFF)":bool=TRUE
  in  "Trap 1 (ON/OFF)":bool=TRUE
  in  "Save Calibration":bool
  out "Manipulating Trap":bool
  out "Buffer Status":dbl(slide)=5.172413793103448e-06 scale=0.0..1.0
  out "Overflow (data lost)":bool
  in  "Reset":bool
  out "Data Rate (Hz)":dbl=100000.0 caption="Trap Data Rate (Hz)" format="%#_3p"
  out "Data Period (s)":dbl=1e-05 caption="Trap Data Period (s)" format="%#_6p"
  in  "BD 1 Frequency 1 (MHz)":dbl=70.0 caption="T1 X (MHz)" min=60.0 max=90.0 step=1.0 format="%#_6p"
  in  "BD 1 Frequency 2 (MHz)":dbl=90.0 caption="T2 X (MHz)" min=60.0 max=90.0 step=1.0 format="%#_6p"
  in  "Round T2 X":bool caption="Round"
  in  "Trap Raster Scan":bool
  out "Raster Scanning...":bool
  in  "Trap Delta (MHz)":dbl=20.0
  in  "Setpoints (V)":cluster{"Set 1":dbl, "Set 2":dbl}={"Set 1"=2.0, "Set 2"=2.0}
  in  "Fish for Tether":bool
  in  "Red FB Setpoint (mV)":dbl=100.0
  in  "Confocal Linescan":bool
  in  "Confocal Image":bool
  in  "Green Laser ON":bool
  in  "AO1":dbl(slide)=0.7905362102114931 caption="Confocal Y (V)" min=0.0 max=10.0 step=0.01 scale=0.0..10.0 scale format="%_1f"
  in  "AO2":dbl(slide)=4.726554155095066 caption="Confocal X (V)" min=0.0 max=10.0 step=0.01 scale=0.0..10.0 scale format="%_1f"
  in  "Green FB Setpoint (mV)":dbl=200.0
  in  "Red Laser ON":bool
  in  "Active Cal":bool
  out "A cal freq (Hz)":dbl=500.0 caption="Freq. (Hz)"
  in  "Laser interlacing mode":enum32{"Laser ON", "Laser OFF", "Interlace"}(radio)=enum."Interlace" caption="Laser interlacing mode (all lasers)"
  in  "Green Intensity % (FB OFF)":dbl=7.0 min=0.0 max=100.0 step=1.0
  in  "Shunt 2":bool caption="Inject Pump 3"
  out "Piezo trap cursor control":cluster{"X":dbl, "Y":dbl}[](graph)
  in  "Scan trap 3 or Fl?":bool=TRUE
  in  "Trap 2 Bead Size (nm)":dbl=1000.0
  in  "Trap 1 Bead Size (nm)":dbl=1000.0
  in  "Dynamic offset\nupdate":bool=TRUE
  in  "Position Label 6":string="0 position (don't change)" caption="6"
  in  "Move to Position 6":bool
  in  "Set Position 6":bool
  in  "Position Label 5":string="central flow spot (UvrD)" caption="5"
  in  "Move to Position":bool
  in  "Position":dbl=1.0 min=1.0 max=10.0 step=1.0
  in  "Set Position":bool
  in  "Saved Stage Positions":dbl[][](array[numeric])=[[1.0, 1.09262, 1.27934, 0.0], [2.0, -0.86772, 0.54946, 0.0311], [3.0, -1.09306, 1.0728, 0.0311], [4.0, 0.19209, 1.30781, 0.0], [5.0, 0.64634, 0.24639, 0.00962], [6.0, 0.0, 0.0, 0.0], [7.0, 0.0, 0.0, 0.0], [8.0, 0.0, 0.0, 0.0], [9.0, 0.0, 0.0, 0.0], [10.0, 0.0, 0.0, 0.0]]
  in  "Move to Position 5":bool
  in  "Position 1 Label":string="Position 1 (lower left)" caption="1"
  in  "Set Position 1":bool
  in  "Set Position 2":bool
  in  "Set Position 3":bool
  in  "Set Position 4":bool
  in  "Move to Position 3":bool
  in  "Move to Position 4":bool
  in  "Move to Position 2":bool
  in  "Move to Position 1":bool
  in  "Position 2 Label":string="Position 2 (upper right)" caption="2"
  in  "Position 3 Label":string="Position 3 (lower right)" caption="3"
  in  "Position 4 Label":string="Experiment position" caption="4"
  in  "Set Position 5":bool
  out "Stage Control Serial Error":errorcluster
  in  "y nudge increment (um":dbl=0.5
  in  "-y":bool
  in  "+y":bool
  in  "x nudge increment (um)":dbl=0.5
  in  "-x":bool
  in  "+x":bool
  in  "-z":bool
  in  "+z":bool
  in  "z nudge increment (um)":dbl=0.5
  in  "Pressure Pump Voltage (+/-10V)":dbl
  in  "Use Harvard pumps\nfor beads (else Chemyx)":bool=TRUE
  in  "Tab Control 9":T13(tab)
  in  "Shunt switch off time (s)":i32
  in  "Auto switch off shunt?":bool
  in  "Force FB at end of shunt?":bool
  in  "Display On P3":bool caption="Display On"
  in  "Normal Flow Rate (ul/h) P3":dbl=800.0 caption="Normal Flow Rate (ul/h)"
  out "Flushing P3":bool caption="Flushing"
  in  "Retract Vol 1 (uL)":dbl=250.0 caption="Volume (uL)"
  in  "Retract Vol 3 (uL)":dbl=250.0 caption="Volume (uL)"
  in  "Retract Rate (uL/m)":dbl=2000.0
  in  "Retract Pump 1":bool
  in  "Retract Pump 3":bool
  in  "Stop Flow":bool
  in  "Start Flow":bool
  in  "Flush Sample":bool
  in  "Volume (uL)":dbl=100.0
  in  "Flush rate (uL/m)":dbl=100.0
  in  "Flow rate (uL/h)":dbl=100.0
  in  "Clear Volume":bool caption="Clear Infused Volume"
  in  "Flush Pump 3":bool
  in  "Volume (uL) P3":dbl=150.0 caption="Volume (uL)"
  in  "Flush rate (uL/m) P3":dbl=100.0 caption="Rate (uL/m)"
  out "Flushing P1":bool caption="Flushing"
  in  "Volume (uL) P1":dbl=100.0 caption="Volume (uL)"
  in  "Flush rate (uL/m) P1":dbl=100.0 caption="Rate (uL/m)"
  in  "Normal Flow Rate (ul/h) P1":dbl=600.0 caption="Normal Flow Rate (ul/h)"
  in  "Flush Pump 1":bool